vi "Main.vi"() -> ()   [LabVIEW 2020]
uses:
  System.Windows.Forms
  Global_Variable/Global.vi
  Database/Global1.vi
  <userlib>/_MGI/Menu Building/MenuTypes/MenuStrip/MGI_MenuStrip.lvclass
  <userlib>/_MGI/Menu Building/MenuItemStatusChange/MGI_MenuItemStatusChange.lvclass
  Libraries/S7/S7.lvlib
panel:
  out "检测结果：":string
  out "条码状态":string
  out "客户软件版本号":string
  in  "Andon":enum32{"未选择", "缺料报警", "质量报警", "故障报警"}(radio)
  out "PLC":bool
  in  "菜单":refnum<k24>(container)
  in  "Result":string[][](table)
  out "逆向空载":bool
  out "试验计时":u16
  out "产品编号":string
  out "生产数量":i32
  out "合格数量":i32
  out "userStatus":string caption="用户状态"
  out "userName":string caption="用户名"
  out "connectionMode":string caption="联机类型"
  out "产品型号":string
  out "功能":bool
  out "空载":bool
  out "振动NVH":bool
  out "磨合":bool
  out "备用试验2":bool
  out "传感器特性":bool
  out "电流特性":bool
  out "力特性":bool
  in  "更换产品":refnum<vi>
  out "提示信息":string
  out "错误":bool
  out "时间字符串":string
  out "日期字符串":string
  out "自动":bool
  # "总成检验"
  # "工艺流程"
  # "试验项目"
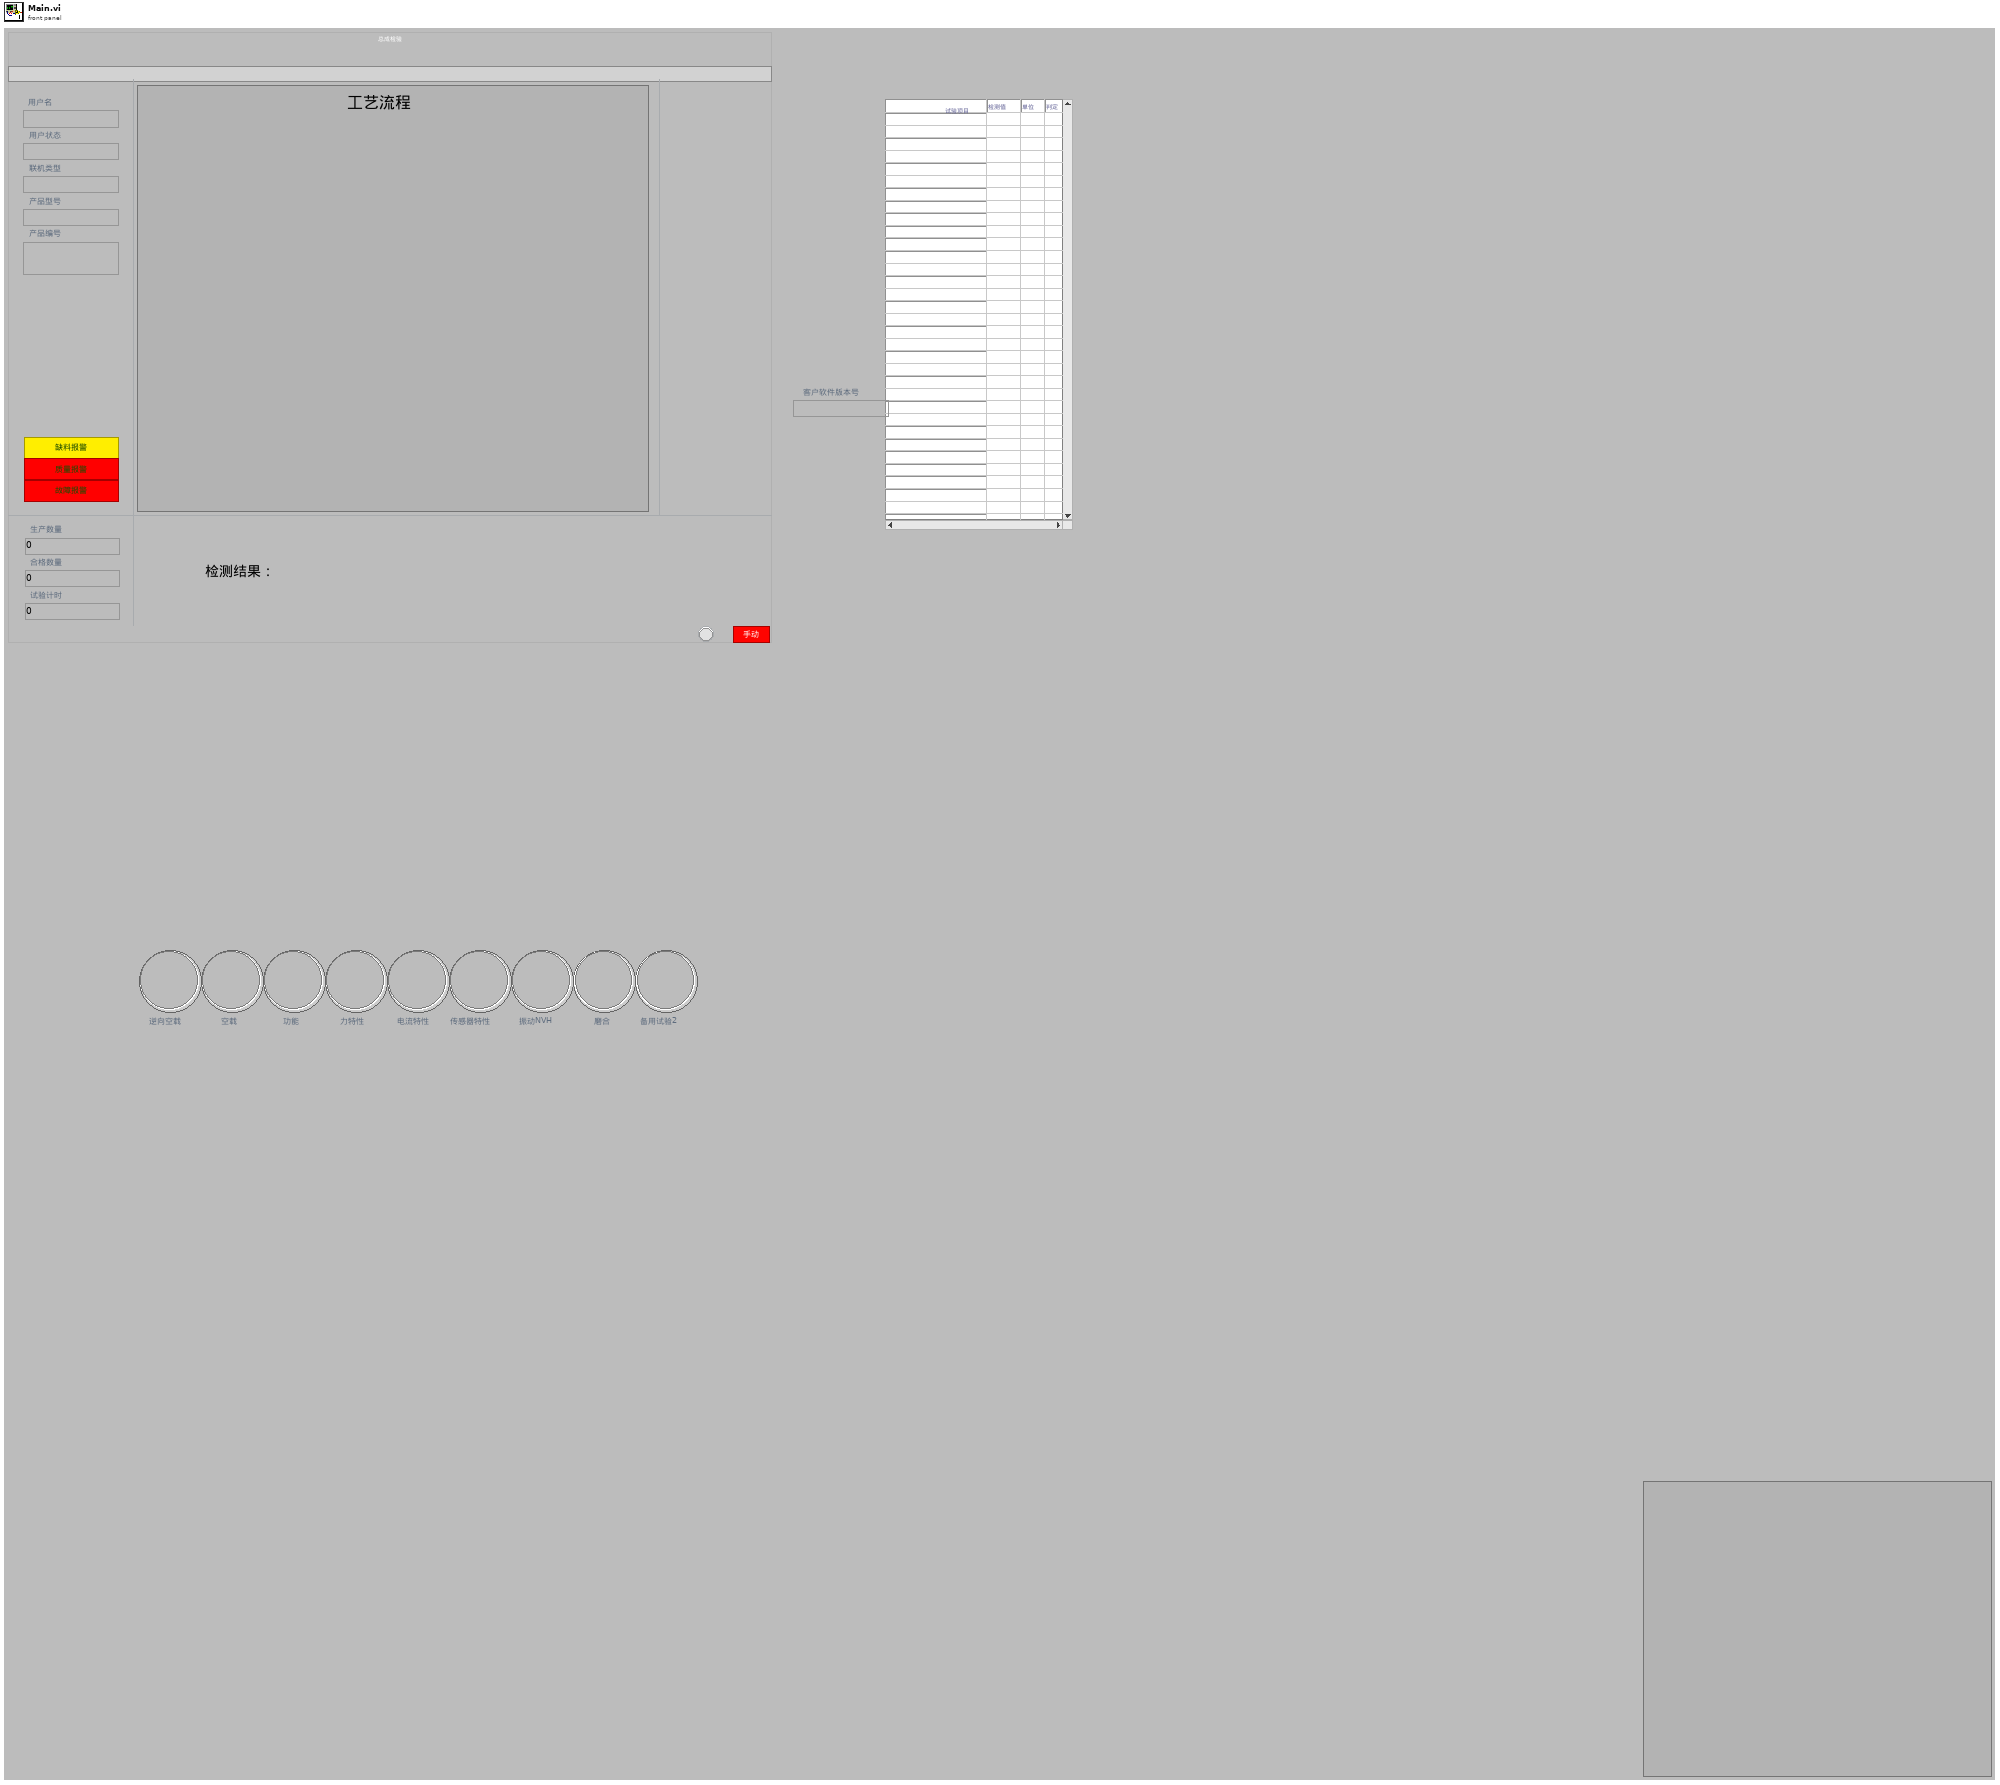
[diagram p1: front panel]
types:
  T1 = typedef "S7.lvlib/Broadcast Events--cluster.ctl" = cluster{"Module Did Init":refnum<user-event>, "Status Updated":refnum<user-event>, "Error Reported":refnum<user-event>, "Module Did Stop":refnum<user-event>, "Update Module Execution Status":refnum<user-event>}
  T2 = enum32{"空载", "功能", "力特性", "电流特性", "传感器特性", "逆向空载", "磨合", "振动NVH"}
  T3 = enum32{"Invalid", "Standard", "Closed", "Hidden", "Minimized", "Maximized"}
  T4 = cluster{"设备名称":string, "操作人员":string, "设备状态":enum16{"设备离线", "设备正常", "设备缺料", "设备故障", "质量报警"}, "附加信息":string}
  T5 = enum32{"invalid app kind", "Development System", "Run Time System", "Student Edition", "Embedded LabVIEW", "Evaluation", "Custom"}
  T6 = cluster{"用户编号":string, "用户名":string, "用户密码(密文)":string, "用户权限":string}
  T7 = cluster{"Core":cluster{"Current VI Reference":refnum<vi>, "Close Panel on Exit?":bool}, "Your Boolean data":bool, "Your string data":string}
  T8 = cluster{"Current VI Reference":refnum<vi>, "Close Panel on Exit?":bool}
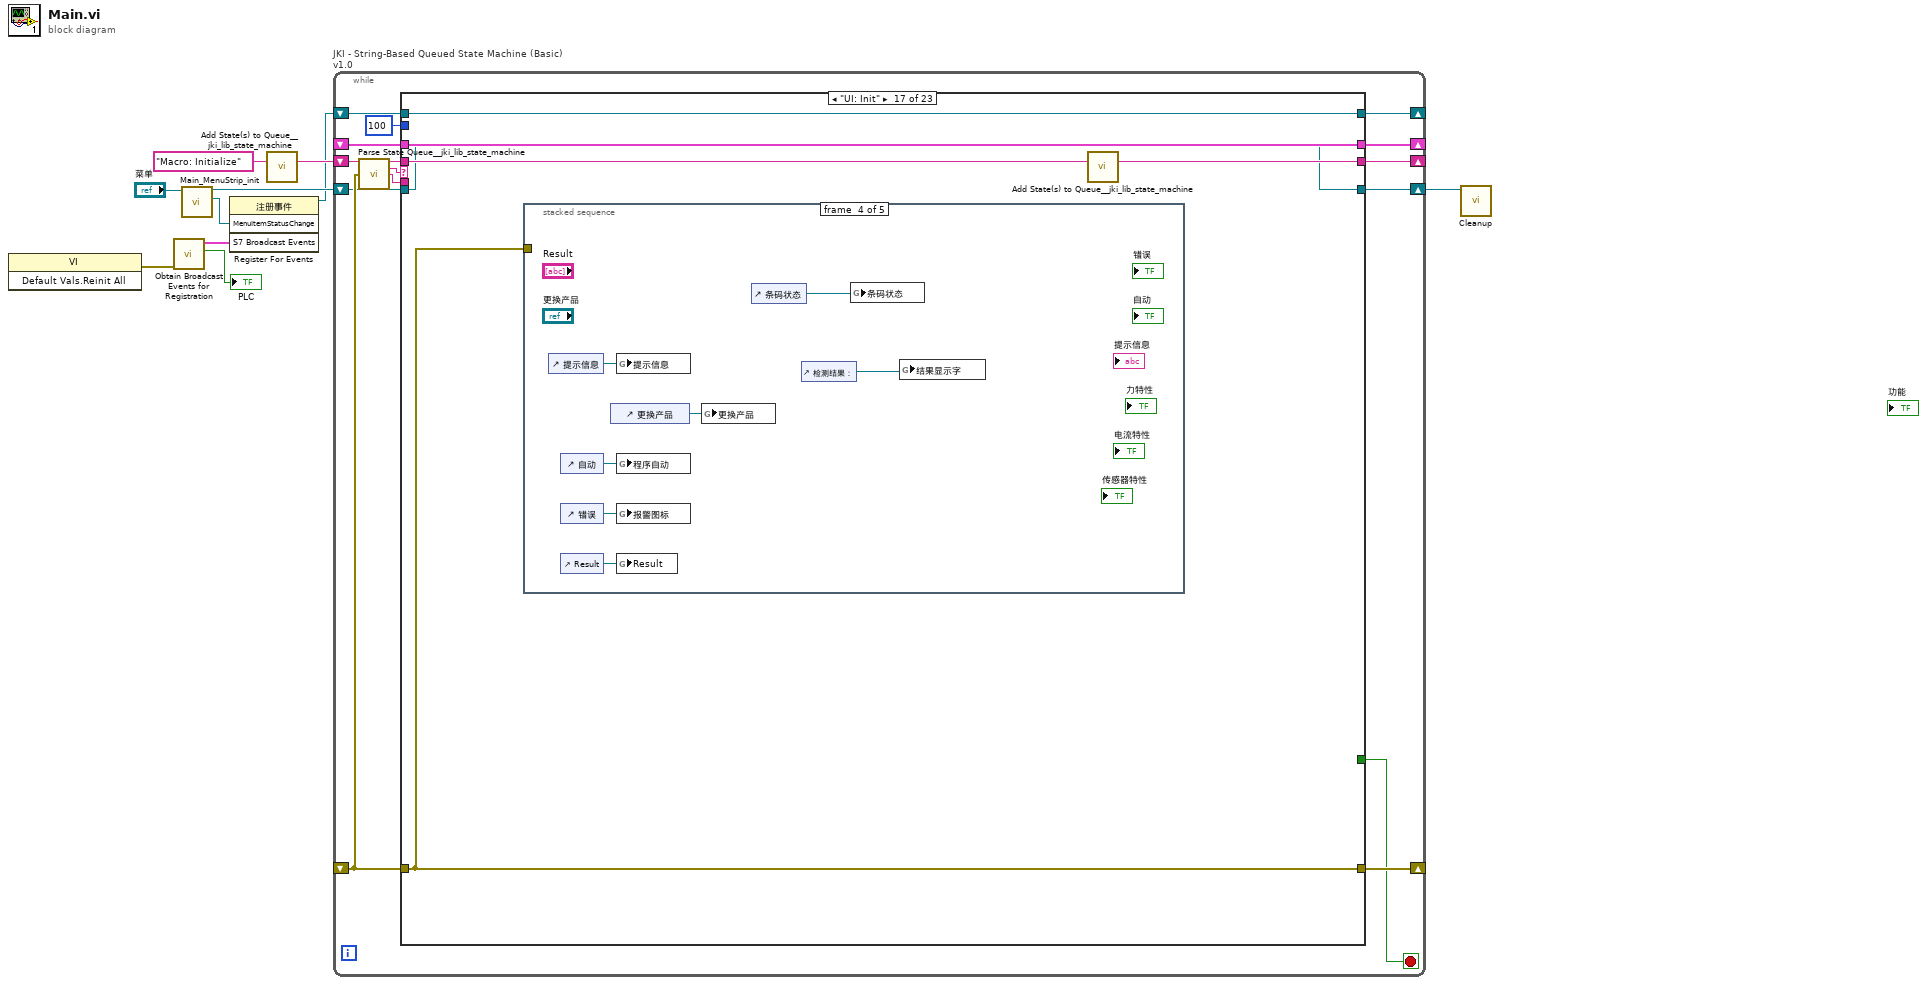
[diagram p0: block diagram]
diagram:
  n1 = invoke class="VI" method="Default Vals.Reinit All"() -> (error out=w3:errorcluster)  [unwired: 3 in, 2 out]
  n2 = call "Obtain Broadcast Events for Registration.vi"("error in (no error)"=w3) -> ("Already running?"=→"PLC":bool, "S7 Broadcast Events"=w5:T1)  [unwired: 8 in, 1 out]
  n3 = call "Main_MenuStrip_init.vi"("MenuStrip"="菜单") -> ("MenuItemStatusChange"=w2:refnum<user-event>, "Menu out"=w7:refnum<class "MGI_MenuStrip.lvclass">)  [unwired: 9 in]
  n4 = register-events(w2, w5) -> (reference out=w1:refnum<event-registration>)  [unwired: 2 in, 1 out]
  n5 = call <vilib>:"Add State(s) to Queue__jki_lib_state_machine.vi"("State(s) in (\"\")"="Macro: Initialize") -> ("States Out"=w10:string)  [unwired: 14 in]
  n6 = while "JKI - String-Based Queued State Machine (Basic) v1.0" {
    shift-right: [w19] -> _
    shift-left: _ -> [w18]
    shift-right: [w21] -> _
    shift-left: _ -> [w16]
    shift-right: [w20] -> _
    shift-left: w10 -> [w22]
    shift-right: [w14] -> w6
    shift-left: w7 -> [w15]
    shift-right: [w12] -> _
    shift-left: w1 -> [w11]
    stop <- w13 stop-if-true
    n7 = call <vilib>:"Parse State Queue__jki_lib_state_machine.vi"("State Queue"=w22, "Error In (no error)"=w16) -> ("Remaining States"=w24:string, "Current State"=w25:string, "Arguments"=w23:string)  [unwired: 11 in]
    n8 = case shown="\"UI: Init\"" w25 {
      selector: w25 -> [_ _ w293 _ _ _ _ _ _ _ _ _ _ _ _ _ _ _ _ _ _ _ _]
      tunnel: w24 -> [w36 w290 w297 w317 w325 w333 w339 w343 w349 w355 w361 w370 w380 w388 w394 w401 w425 w453 w461 w474 w502 w509 w522]
      tunnel: w23 -> [_ _ _ _ _ _ _ _ _ _ _ _ _ _ _ _ _ _ w456 w468 _ _ _]
      tunnel: w18 -> [w34 w287 w295 w308 w322 w331 w336 w344 w352 w358 w364 w367 _ w383 w391 w399 w423 w450 w459 w470 w499 w506 w519]
      tunnel: [w33 w288 w299 w314 errorcluster {"status"=FALSE, "code"=0, "source"=""} ("error out") w330 w337 w341 w347 w354 w360 w368 w377 w384 w392 w398 w421 w451 w457 w471 w500 w507 w520] -> w21
      tunnel: w16 -> [w32 w288 w298 w314 w321 w330 w337 w341 w348 w354 w360 w368 w377 w385 w392 w395 w421 w451 w458 w472 w500 w507 w520]
      tunnel: [w35 w289 w296 w316 w324 w332 w338 w343 w350 w356 w362 w369 w379 w387 w393 w400 w424 w452 w460 w473 w501 w508 w521] -> w20
      tunnel: [w31 w287 w295 w315 w322 w331 w336 w344 w352 w358 w364 w367 w378 w383 w391 w399 w423 w450 w459 w470 w499 w506 w519] -> w19
      tunnel: 100 ("Timeout") -> [w30 _ _ _ _ _ _ _ _ _ _ _ _ _ _ _ _ _ _ _ _ _ _]
      tunnel: w15 -> [w29 w286 w292 w305 w319 w329 w335 w342 w351 w357 w363 w366 w372 w382 w390 w397 w422 w449 w455 w467 w498 w504 w512]
      tunnel: [w28 w286 w292 w305 w319 w329 w335 w342 w351 w357 w363 w366 w372 w382 w390 w397 w422 w449 w455 w467 w498 w504 w512] -> w14
      tunnel: [_ _ _ _ _ TRUE _ _ _ _ _ _ _ _ _ _ _ _ _ _ _ _ _] -> w13
      tunnel: [w26 w285 w291 w304 w318 w327 w334 w345 w346 w353 w359 w365 w373 w381 w389 w396 w420 w446 w454 w466 w497 w503 w511] -> w12
      tunnel: w11 -> [w27 w285 w291 w304 w318 w327 w334 w345 w346 w353 w359 w365 w373 w381 w389 w396 w420 w446 w454 w466 w497 w503 w511]
      frame "", "Event Structure", "Idle" {
        n9 = event shown="[0] 超时" {
          selector: w27 -> [w40 w63 w80 w91 w159 w166 w173 w180 w196 w207 w214 w223 _]
          dyn-events: [w40 w63 w79 w91 w159 w166 w173 w180 w196 w207 w214 w223 _] -> w26
          timeout: w30 -> [_ _ _ _ _ _ _ _ _ _ _ _ _]
          tunnel: w36 -> [w48 w66 w89 w100 w160 w167 w176 w183 w193 w211 w221 w225 w275]
          tunnel: [w47 w65 w89 w98 w161 w168 w177 w184 w194 w212 w220 w226 w275] -> w35
          tunnel: w34 -> [w46 w67 w90 w99 w163 w171 w178 w185 w195 w213 w218 w228 w276]
          tunnel: [w41 w64 w81 w101 w164 w169 w174 w186 w191 w210 w219 w227 w273] -> w33
          tunnel: w32 -> [w41 w64 w82 w101 w164 w169 w174 w187 w191 w210 w219 w227 w273]
          tunnel: [w46 w67 w90 w99 w163 w171 w178 w185 w195 w213 w218 w228 w276] -> w31
          tunnel: w29 -> [w39 _ w88 w94 w162 w170 w175 w182 w192 _ _ _ w274]
          tunnel: [w39 _ w88 w94 w162 w170 w175 w182 w192 _ _ _ w274] -> w28
          event Timeout {
            n10 = event-data() -> ()  [unwired: 1 in, 1 out]
            n11 = disable-structure shown="禁用" {
              frame Disabled {
                n12 = global read "Global.vi" "计时开始"() -> (w50)
                n13 = global read "Global.vi" "软件版本号"() -> (→"客户软件版本号")
                n14 = case shown="真" w50 {
                  frame False {
                    n15 = global write "Global.vi" "计时复位"(TRUE ("计时复位")) -> ()
                  }
                  frame True {
                    n16 = stacked-sequence {
                      frame #0 {
                        n17 = global read "Global.vi" "计时复位"() -> (w52)
                        n18 = call "已用时间"("Reset"=w52) -> ("Elapsed Time (s)"=→"试验计时":dbl)  [unwired: 11 in, 7 out]
                      }
                      frame #1 {
                        n19 = global write "Global.vi" "计时复位"(FALSE ("计时复位")) -> ()
                      }
                    }
                  }
                }
              }
              frame Enabled {
              }
            }
            n20 = Format Date/Time String(time format string (%c)="%H:%M ") -> (date/time string=→"时间字符串":string)  [unwired: 2 in]
            n21 = Format Date/Time String(time format string (%c)="%Y年%m月%d日") -> (date/time string=→"日期字符串":string)  [unwired: 2 in]
            n22 = global read "Global.vi" "产品型号"() -> (w38:string)
            n23 = call <vilib>:"Add State(s) to Queue__jki_lib_state_machine.vi"("State(s) in (\"\")"=w48) -> ("States Out"=w47:string)  [unwired: 14 in]
            n24 = global read "Global1.vi" "工位追溯码"() -> (→"产品编号":string)
            n25 = local write "产品型号"(w38) -> ()
          }
          event "空载", "功能", "力特性", "传感器特性", "电流特性", "振动NVH", "逆向空载", "磨合": Mouse Down {
            w55 = refnum<user-event> refnum items=["空载", "功能", "力特性", "电流特性", "传感器特性", "逆向空载", "磨合", "振动NVH"] ("试验项_Event")
            n26 = event-data() -> ("CtlRef"=w58:refnum<vi>)  [unwired: 1 in]
            n27 = property class="Bool (严格)"(reference=w58) -> ("Label.Text"=w57:string)  [unwired: 1 in, 2 out]
            n28 = vi-ref "A170316-11_Auto.vi"() -> (w61:refnum<vi>)
            n29 = case shown="\"磨合\"" w57 {
              tunnel: [T2."空载" ("事件数据") T2."功能" ("事件数据") T2."力特性" ("事件数据") T2."传感器特性" ("事件数据") T2."电流特性" ("事件数据") T2."逆向空载" ("事件数据") T2."磨合" ("事件数据") T2."振动NVH" ("事件数据")] -> w56
              frame "空载", Default {
              }
              frame "功能" {
              }
              frame "力特性" {
              }
              frame "传感器特性" {
              }
              frame "电流特性" {
              }
              frame "逆向空载" {
              }
              frame "磨合" {
              }
              frame "振动NVH" {
              }
            }
            n30 = invoke class="VI" method="Ctrl Val.Get"(reference=w61, "Control Name"="试验项_Event" ("控件名")) -> ("Get Control Value Variant"=w60:variant)  [unwired: 2 in, 3 out]
            n31 = Variant To Data(type=w55, Variant=w60) -> (data=w59:refnum<user-event>)  [unwired: 1 in, 1 out]
            n32 = Generate User Event(user event=w59, event data cluster=w56) -> ()  [unwired: 2 in, 2 out]
            n33 = call <vilib>:"Add State(s) to Queue__jki_lib_state_machine.vi"("State(s) in (\"\")"=w66) -> ("States Out"=w65:string)  [unwired: 14 in]
          }
          event "PLC": Value Change; "PLC": Mouse Down {
            n34 = event-data() -> ()  [unwired: 1 in, 4 out]
            n35 = call "Start Module.vi"("error in (no error)"=w82) -> ("error out"=w78:errorcluster, "Wait for Event Sync?"=w87:bool, "S7 Broadcast Events"=w86:T1, "Module Was Already Running?"=w85:bool)  [unwired: 7 in]
            n36 = local write "PLC"(w85) -> ()
            n37 = register-events(reference=w80, error in=w78, w86) -> (reference out=w79:refnum<event-registration>, error out=w77:errorcluster)  [unwired: 1 in]
            n38 = call "Synchronize Module Events.vi"("error in (no error)"=w77, "Wait for Event Sync?"=w87) -> ("error out"=w76:errorcluster)  [unwired: 9 in]
            n39 = call "Init S7 Link.vi"("error in (no error)"=w76, "超时"=500, "IP"="192.168.0.121") -> ("error out"=w81:errorcluster)  [unwired: 8 in]
          }
          event User Event {
            n40 = event-data() -> ("StatusChange"=w92:refnum<class "MGI_MenuItemStatusChange.lvclass">)  [unwired: 1 in]
            n41 = call <userlib>:"BasicInfo.vi"("MGI_MenuItemStatusChange in"=w92) -> ("Enabled?"=w95:bool, "Checked?"=w96:bool, "Tag"=w97:string)  [unwired: 7 in, 1 out]
            n42 = case shown="\"设备管理\"" w97 {
              tunnel: w96 -> [_ _ _ _ _ _ _ _ _ _ _ _ _ _ _ _]
              tunnel: w95 -> [_ _ _ _ _ _ _ _ _ _ _ _ _ _ _ _]
              tunnel: [_ _ "S7: Stop\nMacro: Exit" _ _ _ _ _ _ _ _ _ _ _ _ _] -> w93
              frame "假", Default {
              }
              frame "数据库配置" {
                n43 = global read "Global1.vi" "用户信息"() -> (w103:T6)
                n44 = Unbundle By Name(w103) -> ("用户权限"=w102:string)
                n45 = case shown="\"系统管理员\"" w102 {
                  frame Default {
                    n46 = One Button Dialog(message="权限不足！" ("消息")) -> ()  [unwired: 1 in, 1 out]
                  }
                  frame "系统管理员" {
                    n47 = vi-ref "数据库配置.vi"() -> (w106:refnum<vi>)
                    n48 = call "CallVI.vi"("VI引用"=w106, "状态"=T3."Standard") -> ()  [unwired: 11 in, 3 out]
                  }
                }
              }
              frame "退出" {
                n49 = global write "Global.vi" "程序关闭"(TRUE ("程序关闭")) -> ()
                n50 = call "Close_Client.vi"() -> ()  [unwired: 12 in]
              }
              frame "手动控制" {
                n51 = global read "Global1.vi" "用户信息"() -> (w109:T6)
                n52 = Unbundle By Name(w109) -> ("用户权限"=w110:string)
                n53 = case shown="\"班组长\", \"系统管理员\"" w110 {
                  frame Default {
                    n54 = One Button Dialog(message="权限不足！" ("消息")) -> ()  [unwired: 1 in, 1 out]
                  }
                  frame "班组长", "系统管理员" {
                    n55 = vi-ref "A170316-11_IO.vi"() -> (w113:refnum<vi>)
                    n56 = call "CallVI.vi"("VI引用"=w113, "状态"=T3."Standard") -> ()  [unwired: 11 in, 3 out]
                  }
                }
              }
              frame "半自动控制" {
                n57 = disable-structure shown="启用" {
                  frame Disabled {
                    n58 = shared-variable "我的电脑\\Global.lvlib\\操作者权限"() -> (w114:string)  [unwired: 1 in, 1 out]
                    n59 = case shown="\"班组长\", \"系统管理员\"" w114 {
                      frame Default {
                        n60 = One Button Dialog(message="权限不足！" ("消息")) -> ()  [unwired: 1 in, 1 out]
                      }
                      frame "班组长", "系统管理员" {
                        n61 = call "CallVI.vi"("VI引用"=refnum<vi> refnum, "状态"=T3."Maximized") -> ()  [unwired: 11 in, 3 out]
                      }
                    }
                  }
                  frame Enabled {
                    n62 = One Button Dialog(message="当前设备不具备半自动功能！" ("消息")) -> ()  [unwired: 1 in, 1 out]
                  }
                }
              }
              frame "产品管理" {
                n63 = vi-ref "A170316-11_config.vi"() -> (w120:refnum<vi>)
                n64 = call "CallVI.vi"("VI引用"=w120, "状态"=T3."Standard") -> ()  [unwired: 11 in, 3 out]
              }
              frame "系统配置" {
                n65 = global read "Global1.vi" "用户信息"() -> (w122:T6)
                n66 = Unbundle By Name(w122) -> ("用户权限"=w121:string)
                n67 = case shown="\"班组长\", \"操作员\", \"系统管理员\"" w121 {
                  frame Default {
                    n68 = One Button Dialog(message="权限不足！" ("消息")) -> ()  [unwired: 1 in, 1 out]
                  }
                  frame "班组长", "操作员", "系统管理员" {
                    n69 = vi-ref "调试Auto.vi"() -> (w125:refnum<vi>)
                    n70 = call "CallVI.vi"("VI引用"=w125, "状态"=T3."Standard") -> ()  [unwired: 11 in, 3 out]
                  }
                }
              }
              frame "用户管理" {
                n71 = global read "Global1.vi" "用户信息"() -> (w127:T6)
                n72 = Unbundle By Name(w127) -> ("用户权限"=w126:string)
                n73 = case shown="\"系统管理员\"" w126 {
                  frame Default {
                    n74 = One Button Dialog(message="权限不足！" ("消息")) -> ()  [unwired: 1 in, 1 out]
                  }
                  frame "系统管理员" {
                    n75 = vi-ref "User_manager.vi"() -> (w130:refnum<vi>)
                    n76 = call "CallVI.vi"("VI引用"=w130, "状态"=T3."Standard") -> ()  [unwired: 11 in, 3 out]
                  }
                }
              }
              frame "编码规则" {
                n77 = global read "Global1.vi" "用户信息"() -> (w132:T6)
                n78 = Unbundle By Name(w132) -> ("用户权限"=w131:string)
                n79 = case shown="\"班组长\", \"工艺管理员\", \"系统管理员\"" w131 {
                  frame Default {
                    n80 = One Button Dialog(message="权限不足！" ("消息")) -> ()  [unwired: 1 in, 1 out]
                  }
                  frame "班组长", "工艺管理员", "系统管理员" {
                    n81 = vi-ref "编码规则设置.vi"() -> (w135:refnum<vi>)
                    n82 = call "CallVI.vi"("VI引用"=w135, "状态"=T3."Standard") -> ()  [unwired: 11 in, 3 out]
                  }
                }
              }
              frame "易损件管理" {
                n83 = vi-ref "易损件管理.vi"() -> (w137:refnum<vi>)
                n84 = call "CallVI.vi"("VI引用"=w137, "状态"=T3."Standard") -> ()  [unwired: 11 in, 3 out]
              }
              frame "物料批次管理" {
                n85 = vi-ref "批次管理.vi"() -> (w139:refnum<vi>)
                n86 = call "CallVI.vi"("VI引用"=w139, "状态"=T3."Standard") -> ()  [unwired: 11 in, 3 out]
              }
              frame "报表" {
                n87 = call "文件对话框"("start path"=path "D:/report", "prompt"="打开报表", "pattern (all files)"="*.doc;*.docx", "pattern label"="Word 文档") -> ("selected path"=w140:path, "error out"=w141:errorcluster)  [unwired: 8 in, 2 out]
                n88 = case shown="无错误" w141 {
                  selector: w141 -> [w147 w149]
                  tunnel: w140 -> [w148 _]
                  frame No Error {
                    w146 = 1 items=["Normal", "Maximize", "Minimize"] ("cpubbs_WindowState")
                    n89 = call "Open_Word.vi"("File Path"=w148, "cpubbs_WindowState"=w146, "错误输入（无错误）"=w147) -> ()  [unwired: 12 in, 1 out]
                  }
                  frame Error {
                    n90 = call <vilib>:"Clear Errors.vi"("error in (no error)"=w149) -> ()  [unwired: 5 in, 2 out]
                  }
                }
              }
              frame "报警信息" {
                n91 = vi-ref "报警信息.vi"() -> (w151:refnum<vi>)
                n92 = call "CallVI.vi"("VI引用"=w151, "状态"=T3."Standard") -> ()  [unwired: 11 in, 3 out]
              }
              frame "设备管理" {
                n93 = vi-ref "注册设备.vi"() -> (w153:refnum<vi>)
                n94 = call "CallVI.vi"("VI引用"=w153, "状态"=T3."Standard") -> ()  [unwired: 11 in, 3 out]
              }
              frame "关于" {
                n95 = vi-ref "About.vi"() -> (w155:refnum<vi>)
                n96 = call "CallVI.vi"("VI引用"=w155, "状态"=T3."Standard") -> ()  [unwired: 11 in, 3 out]
              }
              frame "操作演示" {
                n97 = call <vilib>:"Application Directory.vi"() -> ("Application Directory"=w158:path)
                n98 = Build Path(base path=w158, name or relative path="操作演示" ("名称或相对路径")) -> (appended path=w157:path)
                n99 = call "自动播放ppt.vi"("路径"=w157) -> ()  [unwired: 10 in, 1 out]
              }
            }
            n100 = call <vilib>:"Add State(s) to Queue__jki_lib_state_machine.vi"("State(s) in (\"\")"=w100, "State(s) at Back (\"\")"=w93) -> ("States Out"=w98:string)  [unwired: 13 in]
          }
          event User Event {
            n101 = event-data() -> ("Init?"=w165:bool)  [unwired: 1 in, 1 out]
            n102 = local write "PLC"(w165) -> ()
            n103 = call <vilib>:"Add State(s) to Queue__jki_lib_state_machine.vi"("State(s) in (\"\")"=w160) -> ("States Out"=w161:string)  [unwired: 14 in]
          }
          event User Event {
            n104 = event-data() -> ("Running?"=w172:bool)  [unwired: 1 in]
            n105 = local write "PLC"(w172) -> ()
            n106 = call <vilib>:"Add State(s) to Queue__jki_lib_state_machine.vi"("State(s) in (\"\")"=w167) -> ("States Out"=w168:string)  [unwired: 14 in]
          }
          event User Event {
            n107 = event-data() -> ()  [unwired: 1 in, 7 out]
            n108 = local write "PLC"(FALSE ("PLC")) -> ()
            n109 = call <vilib>:"Add State(s) to Queue__jki_lib_state_machine.vi"("State(s) in (\"\")"=w176) -> ("States Out"=w177:string)  [unwired: 14 in]
          }
          event User Event {
            n110 = event-data() -> ("Error"=w188:errorcluster)  [unwired: 1 in]
            n111 = Merge Errors(w188, w187) -> (w186:errorcluster)
            n112 = disable-structure shown="禁用" {
              disable-tunnel: ["S7: Stop\nS7: Initialize\nIdle" _] -> w181
              frame Disabled {
              }
              frame Enabled {
              }
            }
            n113 = call <vilib>:"Add State(s) to Queue__jki_lib_state_machine.vi"("State(s) in Front (\"\")"=w181, "State(s) in (\"\")"=w183) -> ("States Out"=w184:string)  [unwired: 13 in]
          }
          event "自动": Mouse Down {
            n114 = event-data() -> ()  [unwired: 1 in, 1 out]
            n115 = local read "自动"() -> (w190:bool)
            n116 = case shown="假" w190 {
              frame False {
                n117 = global read "Global.vi" "设备状态"() -> (w197:i32)
                n118 = case shown="5" w197 {
                  frame 0, Default {
                    n119 = One Button Dialog(message="请复位！" ("消息")) -> ()  [unwired: 1 in, 1 out]
                  }
                  frame 5 {
                    n120 = vi-ref "A170316-11_Auto.vi"() -> (w201:refnum<vi>)
                    n121 = invoke class="VI" method="Ctrl Val.Set"(reference=w201, "Control Name"="STEP" ("控件名"), "Value"="初始化" ("控件名")) -> ()  [unwired: 2 in, 5 out]